vi "生产者消费者.vi"() -> ()   [LabVIEW 2013] (continued)
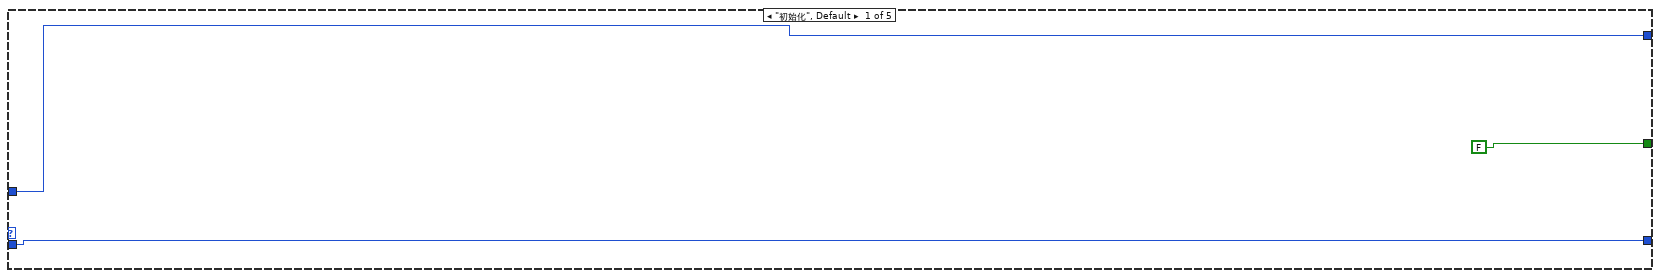
[diagram p2: hidden frame]
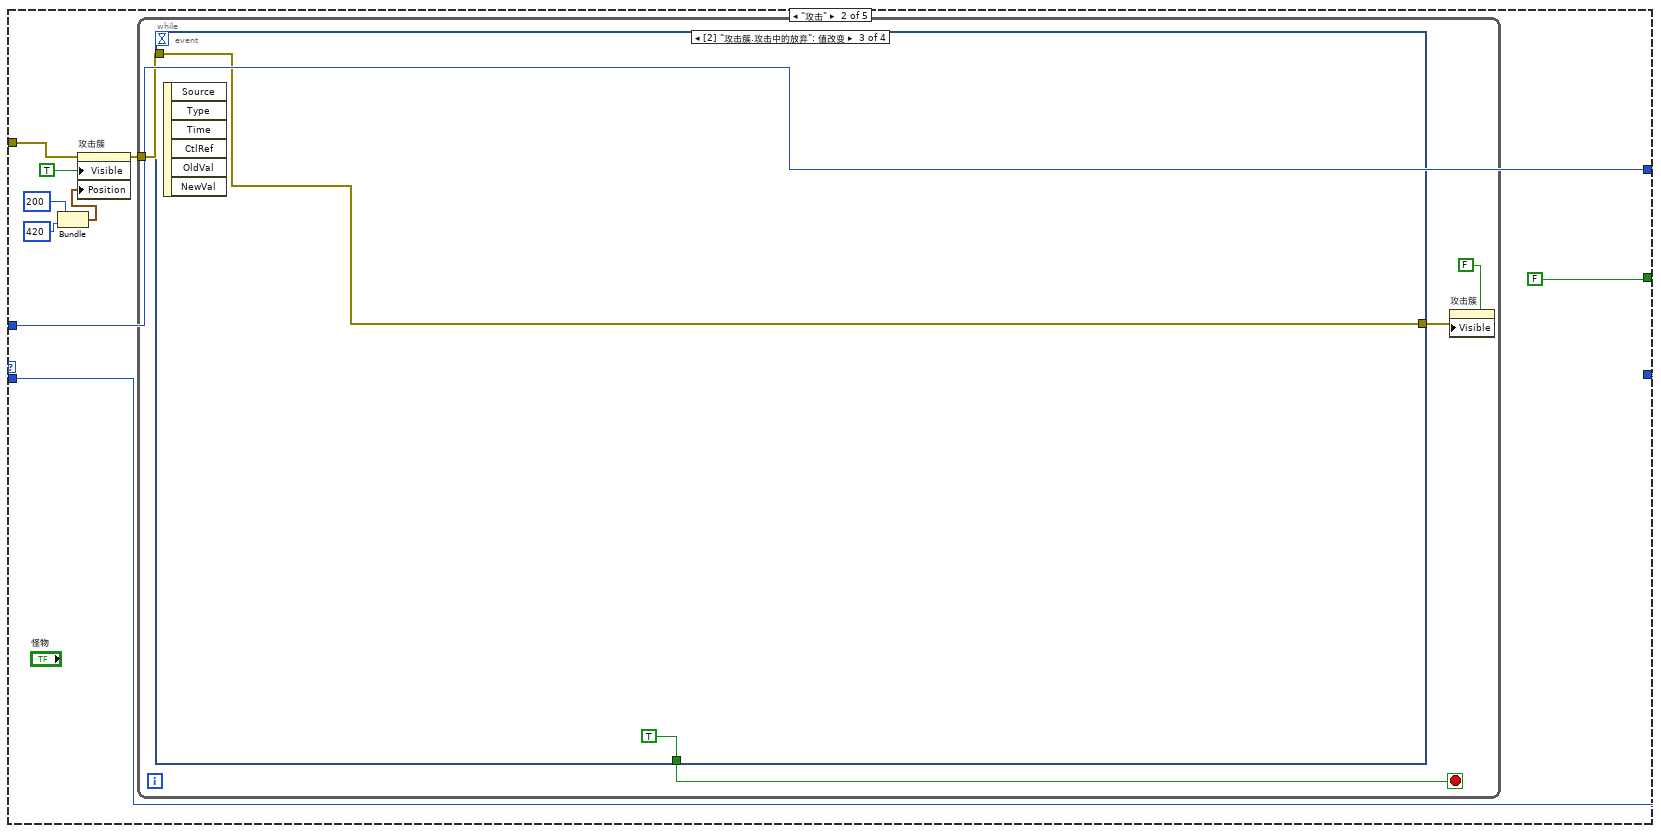
[diagram p3: hidden frame]
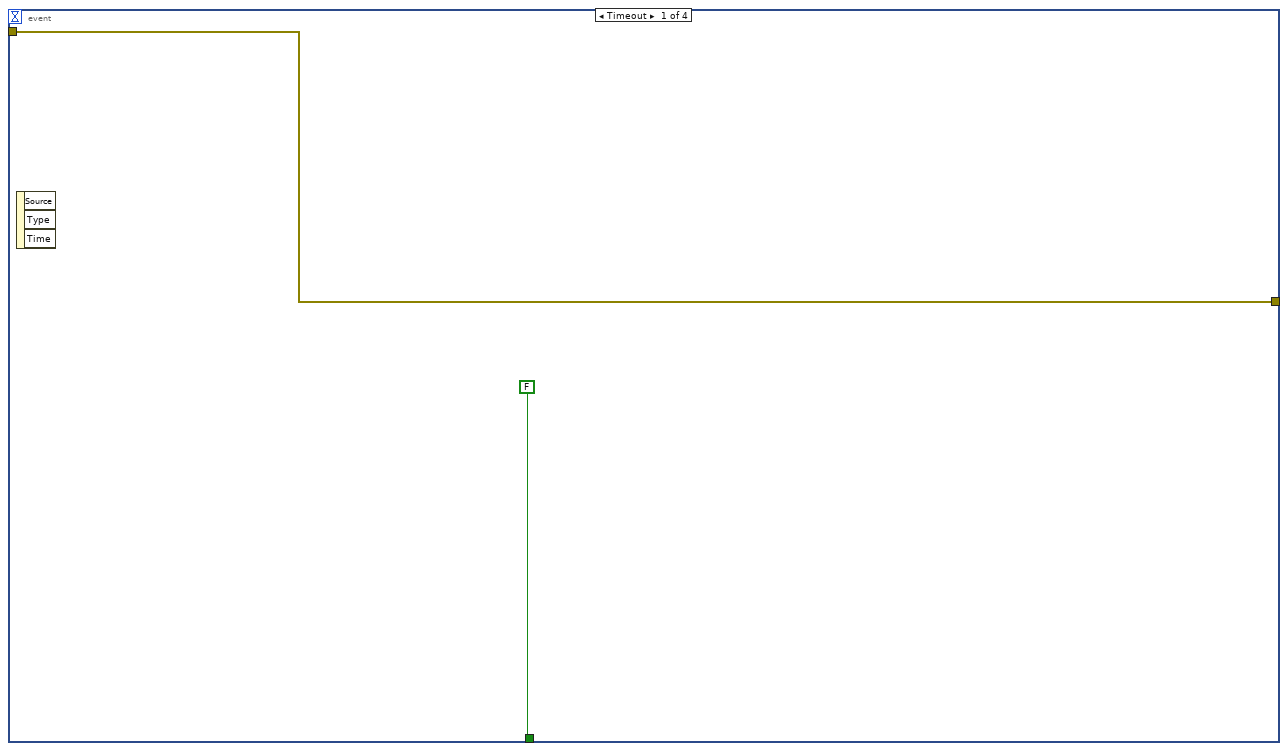
[diagram p4: hidden frame]
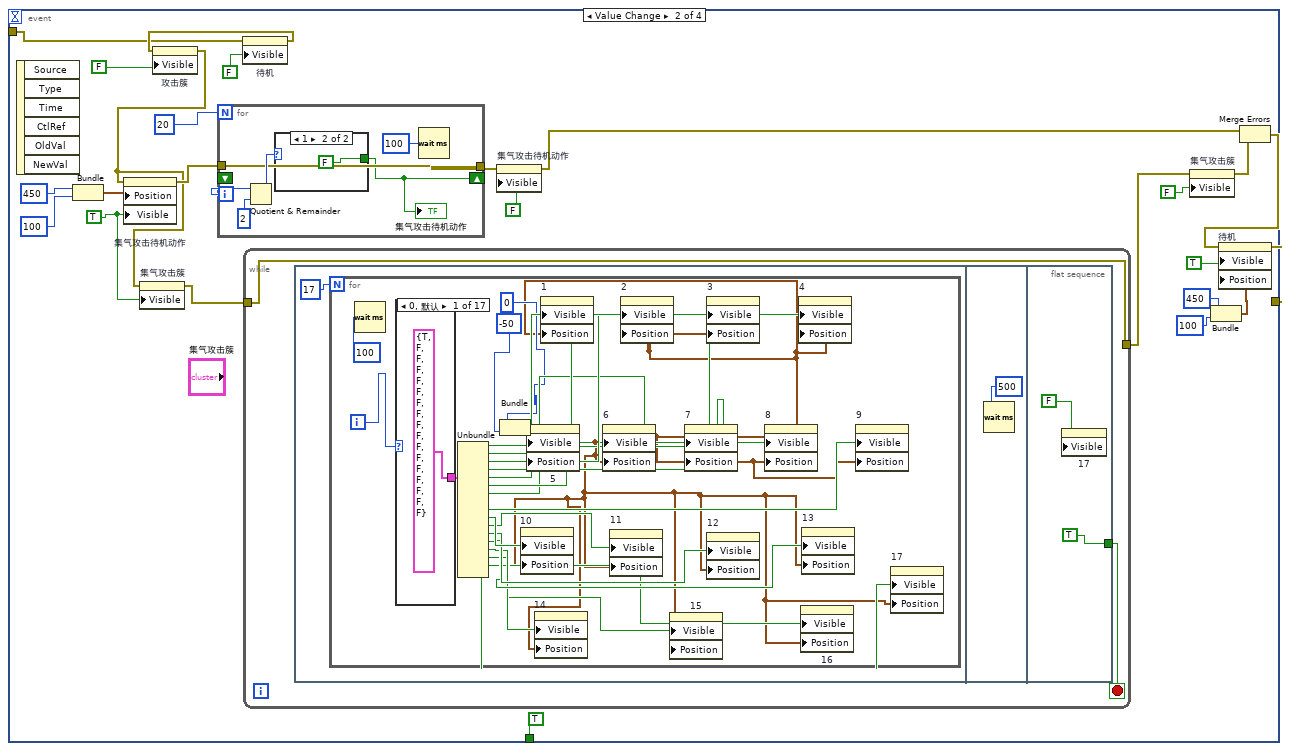
[diagram p5: hidden frame]
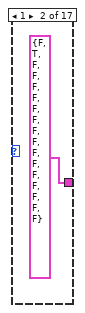
[diagram p6: hidden frame]
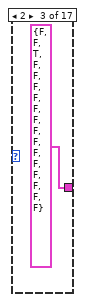
[diagram p7: hidden frame]
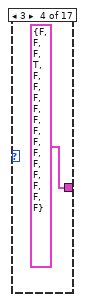
[diagram p8: hidden frame]
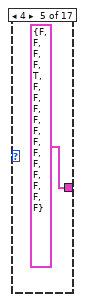
[diagram p9: hidden frame]
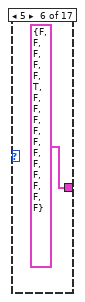
[diagram p10: hidden frame]
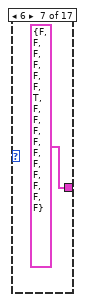
[diagram p11: hidden frame]
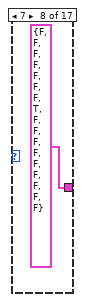
[diagram p12: hidden frame]
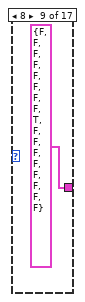
[diagram p13: hidden frame]
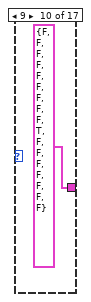
[diagram p14: hidden frame]
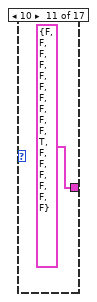
[diagram p15: hidden frame]
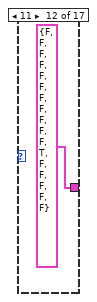
[diagram p16: hidden frame]
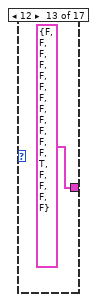
[diagram p17: hidden frame]
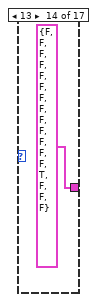
[diagram p18: hidden frame]
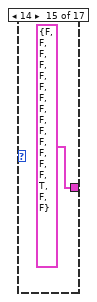
[diagram p19: hidden frame]
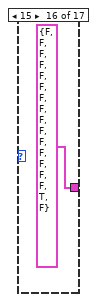
[diagram p20: hidden frame]
                      }
                      frame #2 {
                        n118 = property on="确定按钮" class="Bool"("Visible"=FALSE) -> ()  [unwired: 2 in, 2 out]
                        n119 = property on="15" class="Bool"("Visible"=FALSE) -> ()  [unwired: 2 in, 2 out]
                      }
                    }
                  }
                  n120 = property on="火爪术簇" class="Clust"(error in=w187, "Visible"=FALSE ("可见")) -> ()  [unwired: 1 in, 2 out]
                }
                event "仙术簇.凝冰术": Value Change {
                  n121 = event-data() -> ()  [unwired: 1 in, 6 out]
                  n122 = Bundle(0, 0) -> (w248:cluster{i32, i32})  [unwired: 1 in]
                  n123 = property on="仙术簇" class="Clust"(error in=w251, "Visible"=FALSE) -> (error out=w254:errorcluster)  [unwired: 1 in, 1 out]
                  n124 = property on="待机" class="Bool"(error in=w254, "Visible"=TRUE) -> (error out=w252:errorcluster)  [unwired: 1 in, 1 out]
                  n125 = property on="凝冰术簇" class="Clust"(error in=w252, "Visible"=TRUE, "Position"=w248) -> (error out=w245:errorcluster)  [unwired: 1 in, 1 out]
                  n126 = while {
                    tunnel: w245 -> [w257]
                    tunnel: [w257] -> w244
                    stop <- w258 stop-if-true
                    n127 = flat-sequence {
                      tunnel: [TRUE] -> w258
                      frame #0 {
                        n128 = for {
                          N: 15 -> [_]
                          i -> [w270]
                          n129 = Wait (ms)(milliseconds to wait=100) -> ()  [unwired: 1 out]
                          n130 = case shown="14" w270 {
                            tunnel: [T3 {"4"=TRUE, "5"=FALSE, "6"=FALSE, "7"=FALSE, "8"=FALSE, "1"=FALSE, "2"=FALSE, "3"=FALSE, "9"=FALSE, "10"=FALSE, "11"=FALSE, "12"=FALSE, "13"=FALSE, "14"=FALSE, "15"=FALSE, "确定按钮"=FALSE} ("簇") T3 {"4"=FALSE, "5"=TRUE, "6"=FALSE, "7"=FALSE, "8"=FALSE, "1"=FALSE, "2"=FALSE, "3"=FALSE, "9"=FALSE, "10"=FALSE, "11"=FALSE, "12"=FALSE, "13"=FALSE, "14"=FALSE, "15"=FALSE, "确定按钮"=FALSE} ("簇") T3 {"4"=FALSE, "5"=FALSE, "6"=TRUE, "7"=FALSE, "8"=FALSE, "1"=FALSE, "2"=FALSE, "3"=FALSE, "9"=FALSE, "10"=FALSE, "11"=FALSE, "12"=FALSE, "13"=FALSE, "14"=FALSE, "15"=FALSE, "确定按钮"=FALSE} ("簇") T3 {"4"=FALSE, "5"=FALSE, "6"=FALSE, "7"=TRUE, "8"=FALSE, "1"=FALSE, "2"=FALSE, "3"=FALSE, "9"=FALSE, "10"=FALSE, "11"=FALSE, "12"=FALSE, "13"=FALSE, "14"=FALSE, "15"=FALSE, "确定按钮"=FALSE} ("簇") T3 {"4"=FALSE, "5"=FALSE, "6"=FALSE, "7"=FALSE, "8"=TRUE, "1"=FALSE, "2"=FALSE, "3"=FALSE, "9"=FALSE, "10"=FALSE, "11"=FALSE, "12"=FALSE, "13"=FALSE, "14"=FALSE, "15"=FALSE, "确定按钮"=FALSE} ("簇") T3 {"4"=FALSE, "5"=FALSE, "6"=FALSE, "7"=FALSE, "8"=FALSE, "1"=TRUE, "2"=FALSE, "3"=FALSE, "9"=FALSE, "10"=FALSE, "11"=FALSE, "12"=FALSE, "13"=FALSE, "14"=FALSE, "15"=FALSE, "确定按钮"=FALSE} ("簇") T3 {"4"=FALSE, "5"=FALSE, "6"=FALSE, "7"=FALSE, "8"=FALSE, "1"=FALSE, "2"=TRUE, "3"=FALSE, "9"=FALSE, "10"=FALSE, "11"=FALSE, "12"=FALSE, "13"=FALSE, "14"=FALSE, "15"=FALSE, "确定按钮"=FALSE} ("簇") T3 {"4"=FALSE, "5"=FALSE, "6"=FALSE, "7"=FALSE, "8"=FALSE, "1"=FALSE, "2"=FALSE, "3"=TRUE, "9"=FALSE, "10"=FALSE, "11"=FALSE, "12"=FALSE, "13"=FALSE, "14"=FALSE, "15"=FALSE, "确定按钮"=FALSE} ("簇") T3 {"4"=FALSE, "5"=FALSE, "6"=FALSE, "7"=FALSE, "8"=FALSE, "1"=FALSE, "2"=FALSE, "3"=FALSE, "9"=TRUE, "10"=FALSE, "11"=FALSE, "12"=FALSE, "13"=FALSE, "14"=FALSE, "15"=FALSE, "确定按钮"=FALSE} ("簇") T3 {"4"=FALSE, "5"=FALSE, "6"=FALSE, "7"=FALSE, "8"=FALSE, "1"=FALSE, "2"=FALSE, "3"=FALSE, "9"=FALSE, "10"=TRUE, "11"=FALSE, "12"=FALSE, "13"=FALSE, "14"=FALSE, "15"=FALSE, "确定按钮"=FALSE} ("簇") T3 {"4"=FALSE, "5"=FALSE, "6"=FALSE, "7"=FALSE, "8"=FALSE, "1"=FALSE, "2"=FALSE, "3"=FALSE, "9"=FALSE, "10"=FALSE, "11"=TRUE, "12"=FALSE, "13"=FALSE, "14"=FALSE, "15"=FALSE, "确定按钮"=FALSE} ("簇") T3 {"4"=FALSE, "5"=FALSE, "6"=FALSE, "7"=FALSE, "8"=FALSE, "1"=FALSE, "2"=FALSE, "3"=FALSE, "9"=FALSE, "10"=FALSE, "11"=FALSE, "12"=TRUE, "13"=FALSE, "14"=FALSE, "15"=FALSE, "确定按钮"=FALSE} ("簇") T3 {"4"=FALSE, "5"=FALSE, "6"=FALSE, "7"=FALSE, "8"=FALSE, "1"=FALSE, "2"=FALSE, "3"=FALSE, "9"=FALSE, "10"=FALSE, "11"=FALSE, "12"=FALSE, "13"=TRUE, "14"=FALSE, "15"=FALSE, "确定按钮"=FALSE} ("簇") T3 {"4"=FALSE, "5"=FALSE, "6"=FALSE, "7"=FALSE, "8"=FALSE, "1"=FALSE, "2"=FALSE, "3"=FALSE, "9"=FALSE, "10"=FALSE, "11"=FALSE, "12"=FALSE, "13"=FALSE, "14"=TRUE, "15"=FALSE, "确定按钮"=FALSE} ("簇") T3 {"4"=FALSE, "5"=FALSE, "6"=FALSE, "7"=FALSE, "8"=FALSE, "1"=FALSE, "2"=FALSE, "3"=FALSE, "9"=FALSE, "10"=FALSE, "11"=FALSE, "12"=FALSE, "13"=FALSE, "14"=FALSE, "15"=TRUE, "确定按钮"=FALSE} ("簇")] -> w269
                            frame 0, Default {
                            }
                            frame 1 {
                            }
                            frame 2 {
                            }
                            frame 3 {
                            }
                            frame 4 {
                            }
                            frame 5 {
                            }
                            frame 6 {
                            }
                            frame 7 {
                            }
                            frame 8 {
                            }
                            frame 9 {
                            }
                            frame 10 {
                            }
                            frame 11 {
                            }
                            frame 12 {
                            }
                            frame 13 {
                            }
                            frame 14 {
                            }
                          }
                          n131 = Unbundle(w269) -> ("4"=w282:bool, "5"=w281:bool, "6"=w280:bool, "7"=w279:bool, "8"=w278:bool, "1"=w277:bool, "2"=w265:bool, "3"=w264:bool, "9"=w274:bool, "10"=w273:bool, "11"=w268:bool, "12"=w272:bool, "13"=w262:bool, "14"=w263:bool, "15"=w260:bool)  [unwired: 1 out]
                          n132 = Bundle(50, 0) -> (w271:cluster{i32, i32})  [unwired: 1 in]
                          n133 = property on="确定按钮 10" class="Bool"("Visible"=w273, "Position"=w271) -> ()  [unwired: 2 in, 2 out]
                          n134 = property on="确定按钮 5" class="Bool"("Visible"=w278, "Position"=w271) -> ()  [unwired: 2 in, 2 out]
                          n135 = property on="确定按钮 14" class="Bool"("Visible"=w263, "Position"=w271) -> ()  [unwired: 2 in, 2 out]
                          n136 = property on="确定按钮1" class="Bool"("Visible"=w282, "Position"=w271) -> ()  [unwired: 2 in, 2 out]
                          n137 = property on="确定按钮 6" class="Bool"("Visible"=w277, "Position"=w271) -> ()  [unwired: 2 in, 2 out]
                          n138 = property on="确定按钮 11" class="Bool"("Visible"=w268, "Position"=w271) -> ()  [unwired: 2 in, 2 out]
                          n139 = property on="确定按钮 2" class="Bool"("Visible"=w281, "Position"=w271) -> ()  [unwired: 2 in, 2 out]
                          n140 = property on="确定按钮 15" class="Bool"("Visible"=w260, "Position"=w271) -> ()  [unwired: 2 in, 2 out]
                          n141 = property on="确定按钮 7" class="Bool"("Visible"=w265, "Position"=w271) -> ()  [unwired: 2 in, 2 out]
                          n142 = property on="确定按钮 3" class="Bool"("Visible"=w280, "Position"=w271) -> ()  [unwired: 2 in, 2 out]
                          n143 = property on="确定按钮 12" class="Bool"("Visible"=w272, "Position"=w271) -> ()  [unwired: 2 in, 2 out]
                          n144 = property on="确定按钮 8" class="Bool"("Visible"=w264, "Position"=w271) -> ()  [unwired: 2 in, 2 out]
                          n145 = Bundle(100, 50) -> (w261:cluster{i32, i32})  [unwired: 1 in]
                          n146 = property on="确定按钮 4" class="Bool"("Visible"=w279, "Position"=w271) -> ()  [unwired: 2 in, 2 out]
                          n147 = property on="确定按钮 13" class="Bool"("Visible"=w262, "Position"=w271) -> ()  [unwired: 2 in, 2 out]
                          n148 = property class="Bool"("Visible"=w260, "Position"=w261) -> ()  [unwired: 2 in, 2 out]
                          n149 = property on="确定按钮 9" class="Bool"("Visible"=w274, "Position"=w271) -> ()  [unwired: 2 in, 2 out]
                        }
                      }
                      frame #1 {
                        n150 = Wait (ms)(milliseconds to wait=500) -> ()  [unwired: 1 out]
                      }
                      frame #2 {
                        n151 = property on="确定按钮 15" class="Bool"("Visible"=FALSE) -> ()  [unwired: 2 in, 2 out]
                        n152 = property class="Bool"("Visible"=FALSE) -> ()  [unwired: 2 in, 2 out]
                      }
                    }
                  }
                  n153 = property on="凝冰术簇" class="Clust"(error in=w244, "Visible"=FALSE ("可见")) -> ()  [unwired: 1 in, 2 out]
                }
                event "仙术簇.疾风术": Value Change {
                  n154 = event-data() -> ()  [unwired: 1 in, 6 out]
                  n155 = Bundle(0, 0) -> (w307:cluster{i32, i32})  [unwired: 1 in]
                  n156 = property on="仙术簇" class="Clust"(error in=w310, "Visible"=FALSE) -> (error out=w313:errorcluster)  [unwired: 1 in, 1 out]
                  n157 = property on="待机" class="Bool"(error in=w313, "Visible"=TRUE) -> (error out=w311:errorcluster)  [unwired: 1 in, 1 out]
                  n158 = property on="疾风术簇" class="Clust"(error in=w311, "Visible"=TRUE, "Position"=w307) -> (error out=w304:errorcluster)  [unwired: 1 in, 1 out]
                  n159 = while {
                    tunnel: w304 -> [w316]
                    tunnel: [w316] -> w303
                    stop <- w317 stop-if-true
                    n160 = flat-sequence {
                      tunnel: [TRUE] -> w317
                      frame #0 {
                        n161 = for {
                          N: 14 -> [_]
                          i -> [w330]
                          n162 = Wait (ms)(milliseconds to wait=100) -> ()  [unwired: 1 out]
                          n163 = case shown="13" w330 {
                            tunnel: [T3 {"4"=TRUE, "5"=FALSE, "6"=FALSE, "7"=FALSE, "8"=FALSE, "1"=FALSE, "2"=FALSE, "3"=FALSE, "9"=FALSE, "10"=FALSE, "11"=FALSE, "12"=FALSE, "13"=FALSE, "14"=FALSE, "15"=FALSE, "确定按钮"=FALSE} ("簇") T3 {"4"=FALSE, "5"=TRUE, "6"=FALSE, "7"=FALSE, "8"=FALSE, "1"=FALSE, "2"=FALSE, "3"=FALSE, "9"=FALSE, "10"=FALSE, "11"=FALSE, "12"=FALSE, "13"=FALSE, "14"=FALSE, "15"=FALSE, "确定按钮"=FALSE} ("簇") T3 {"4"=FALSE, "5"=FALSE, "6"=TRUE, "7"=FALSE, "8"=FALSE, "1"=FALSE, "2"=FALSE, "3"=FALSE, "9"=FALSE, "10"=FALSE, "11"=FALSE, "12"=FALSE, "13"=FALSE, "14"=FALSE, "15"=FALSE, "确定按钮"=FALSE} ("簇") T3 {"4"=FALSE, "5"=FALSE, "6"=FALSE, "7"=TRUE, "8"=FALSE, "1"=FALSE, "2"=FALSE, "3"=FALSE, "9"=FALSE, "10"=FALSE, "11"=FALSE, "12"=FALSE, "13"=FALSE, "14"=FALSE, "15"=FALSE, "确定按钮"=FALSE} ("簇") T3 {"4"=FALSE, "5"=FALSE, "6"=FALSE, "7"=FALSE, "8"=TRUE, "1"=FALSE, "2"=FALSE, "3"=FALSE, "9"=FALSE, "10"=FALSE, "11"=FALSE, "12"=FALSE, "13"=FALSE, "14"=FALSE, "15"=FALSE, "确定按钮"=FALSE} ("簇") T3 {"4"=FALSE, "5"=FALSE, "6"=FALSE, "7"=FALSE, "8"=FALSE, "1"=TRUE, "2"=FALSE, "3"=FALSE, "9"=FALSE, "10"=FALSE, "11"=FALSE, "12"=FALSE, "13"=FALSE, "14"=FALSE, "15"=FALSE, "确定按钮"=FALSE} ("簇") T3 {"4"=FALSE, "5"=FALSE, "6"=FALSE, "7"=FALSE, "8"=FALSE, "1"=FALSE, "2"=TRUE, "3"=FALSE, "9"=FALSE, "10"=FALSE, "11"=FALSE, "12"=FALSE, "13"=FALSE, "14"=FALSE, "15"=FALSE, "确定按钮"=FALSE} ("簇") T3 {"4"=FALSE, "5"=FALSE, "6"=FALSE, "7"=FALSE, "8"=FALSE, "1"=FALSE, "2"=FALSE, "3"=TRUE, "9"=FALSE, "10"=FALSE, "11"=FALSE, "12"=FALSE, "13"=FALSE, "14"=FALSE, "15"=FALSE, "确定按钮"=FALSE} ("簇") T3 {"4"=FALSE, "5"=FALSE, "6"=FALSE, "7"=FALSE, "8"=FALSE, "1"=FALSE, "2"=FALSE, "3"=FALSE, "9"=TRUE, "10"=FALSE, "11"=FALSE, "12"=FALSE, "13"=FALSE, "14"=FALSE, "15"=FALSE, "确定按钮"=FALSE} ("簇") T3 {"4"=FALSE, "5"=FALSE, "6"=FALSE, "7"=FALSE, "8"=FALSE, "1"=FALSE, "2"=FALSE, "3"=FALSE, "9"=FALSE, "10"=TRUE, "11"=FALSE, "12"=FALSE, "13"=FALSE, "14"=FALSE, "15"=FALSE, "确定按钮"=FALSE} ("簇") T3 {"4"=FALSE, "5"=FALSE, "6"=FALSE, "7"=FALSE, "8"=FALSE, "1"=FALSE, "2"=FALSE, "3"=FALSE, "9"=FALSE, "10"=FALSE, "11"=TRUE, "12"=FALSE, "13"=FALSE, "14"=FALSE, "15"=FALSE, "确定按钮"=FALSE} ("簇") T3 {"4"=FALSE, "5"=FALSE, "6"=FALSE, "7"=FALSE, "8"=FALSE, "1"=FALSE, "2"=FALSE, "3"=FALSE, "9"=FALSE, "10"=FALSE, "11"=FALSE, "12"=TRUE, "13"=FALSE, "14"=FALSE, "15"=FALSE, "确定按钮"=FALSE} ("簇") T3 {"4"=FALSE, "5"=FALSE, "6"=FALSE, "7"=FALSE, "8"=FALSE, "1"=FALSE, "2"=FALSE, "3"=FALSE, "9"=FALSE, "10"=FALSE, "11"=FALSE, "12"=FALSE, "13"=TRUE, "14"=FALSE, "15"=FALSE, "确定按钮"=FALSE} ("簇") T3 {"4"=FALSE, "5"=FALSE, "6"=FALSE, "7"=FALSE, "8"=FALSE, "1"=FALSE, "2"=FALSE, "3"=FALSE, "9"=FALSE, "10"=FALSE, "11"=FALSE, "12"=FALSE, "13"=FALSE, "14"=TRUE, "15"=FALSE, "确定按钮"=FALSE} ("簇")] -> w329
                            frame 0, Default {
                            }
                            frame 1 {
                            }
                            frame 2 {
                            }
                            frame 3 {
                            }
                            frame 4 {
                            }
                            frame 5 {
                            }
                            frame 6 {
                            }
                            frame 7 {
                            }
                            frame 8 {
                            }
                            frame 9 {
                            }
                            frame 10 {
                            }
                            frame 11 {
                            }
                            frame 12 {
                            }
                            frame 13 {
                            }
                          }
                          n164 = Unbundle(w329) -> ("4"=w341:bool, "5"=w340:bool, "6"=w339:bool, "7"=w338:bool, "8"=w337:bool, "1"=w336:bool, "2"=w326:bool, "3"=w325:bool, "9"=w333:bool, "10"=w332:bool, "11"=w323:bool, "12"=w322:bool, "13"=w321:bool, "14"=w320:bool)  [unwired: 2 out]
                          n165 = Bundle(50, 0) -> (w331:cluster{i32, i32})  [unwired: 1 in]
                          n166 = property on="确定按钮 10" class="Bool"("Visible"=w332, "Position"=w331) -> ()  [unwired: 2 in, 2 out]
                          n167 = property on="确定按钮 5" class="Bool"("Visible"=w337, "Position"=w331) -> ()  [unwired: 2 in, 2 out]
                          n168 = property on="确定按钮 14" class="Bool"("Visible"=w320, "Position"=w331) -> ()  [unwired: 2 in, 2 out]
                          n169 = property on="确定按钮" class="Bool"("Visible"=w341, "Position"=w331) -> ()  [unwired: 2 in, 2 out]
                          n170 = property on="确定按钮 6" class="Bool"("Visible"=w336, "Position"=w331) -> ()  [unwired: 2 in, 2 out]
                          n171 = property on="确定按钮 11" class="Bool"("Visible"=w323, "Position"=w331) -> ()  [unwired: 2 in, 2 out]
                          n172 = property on="确定按钮 2" class="Bool"("Visible"=w340, "Position"=w331) -> ()  [unwired: 2 in, 2 out]
                          n173 = Compound Arithmetic op=OR(w323, w322, w321, w320) -> (w319:bool)
                          n174 = property on="确定按钮 7" class="Bool"("Visible"=w326, "Position"=w331) -> ()  [unwired: 2 in, 2 out]
                          n175 = property on="确定按钮 3" class="Bool"("Visible"=w339, "Position"=w331) -> ()  [unwired: 2 in, 2 out]
                          n176 = property on="确定按钮 12" class="Bool"("Visible"=w322, "Position"=w331) -> ()  [unwired: 2 in, 2 out]
                          n177 = property on="确定按钮 8" class="Bool"("Visible"=w325, "Position"=w331) -> ()  [unwired: 2 in, 2 out]
                          n178 = Bundle(50, 50) -> (w324:cluster{i32, i32})  [unwired: 1 in]
                          n179 = property on="确定按钮 4" class="Bool"("Visible"=w338, "Position"=w331) -> ()  [unwired: 2 in, 2 out]
                          n180 = property on="确定按钮 13" class="Bool"("Visible"=w321, "Position"=w331) -> ()  [unwired: 2 in, 2 out]
                          n181 = property on="确定按钮 15" class="Bool"("Visible"=w319, "Position"=w324) -> ()  [unwired: 2 in, 2 out]
                          n182 = property on="确定按钮 9" class="Bool"("Visible"=w333, "Position"=w331) -> ()  [unwired: 2 in, 2 out]
                        }
                      }
                      frame #1 {
                        n183 = Wait (ms)(milliseconds to wait=500) -> ()  [unwired: 1 out]
                      }
                      frame #2 {
                        n184 = property on="确定按钮 14" class="Bool"("Visible"=FALSE) -> ()  [unwired: 2 in, 2 out]
                        n185 = property on="确定按钮 15" class="Bool"("Visible"=FALSE) -> ()  [unwired: 2 in, 2 out]
                      }
                    }
                  }
                  n186 = property on="疾风术簇" class="Clust"(error in=w303, "Visible"=FALSE ("可见")) -> ()  [unwired: 1 in, 2 out]
                }
                event "仙术簇.仙术中的放弃": Value Change {
                  n187 = event-data() -> ()  [unwired: 1 in, 6 out]
                  n188 = property on="仙术簇" class="Clust"(error in=w361, "Visible"=FALSE) -> ()  [unwired: 1 in, 2 out]
                }
              }
            }
          }
          frame "物品" {
            w366 = FALSE
            n189 = Bundle(200, 420) -> (w375:cluster{i32, i32})  [unwired: 1 in]
            n190 = property on="物品簇" class="Clust"(error in=w379, "Visible"=TRUE, "Position"=w375) -> (error out=w378:errorcluster)  [unwired: 1 in, 1 out]
            n191 = while {
              tunnel: w378 -> [w386]
              tunnel: w374 -> [w385]
              tunnel: [w382] -> w373
              tunnel: [w384] -> w369
              tunnel: w368 -> [w383]
              tunnel: [w381] -> w367
              stop <- w387 stop-if-true
              n192 = event shown="[1] \"物品簇.止血草\": 鼠标进入" {
                selector: _ -> [_ _ _ _ _ _ _]
                dyn-events: _ -> [_ _ _ _ _ _ _]
                timeout: _ -> [_ _ _ _ _ _ _]
                tunnel: [w390 w392 w407 w416 w429 w440 w444] -> w384
                tunnel: [FALSE FALSE FALSE TRUE TRUE TRUE FALSE] -> w387
                tunnel: w386 -> [w390 w402 w413 w416 w429 w440 w442]
                tunnel: w385 -> [w389 w397 w408 w417 w427 w439 w443]
                tunnel: [w389 w397 w408 w418 w427 w439 w443] -> w382
                tunnel: w383 -> [w388 w396 w406 w415 w428 w437 w441]
                tunnel: [w388 w396 w406 w415 w426 w437 w441] -> w381
                event Timeout {
                  n193 = event-data() -> ()  [unwired: 1 in, 3 out]
                }
                event "物品簇.止血草": Mouse Enter {
                  (unwired) 10
                  n194 = event-data() -> ()  [unwired: 1 in, 4 out]
                  n195 = Bundle(400, 200) -> (w398:cluster{i32, i32})  [unwired: 1 in]
                  n196 = property on="琉璃法珠簇" class="Clust"(error in=w402, "Visible"=TRUE, "Position"=w398) -> (error out=w395:errorcluster)  [unwired: 1 in, 1 out]
                  n197 = flat-sequence {
                    tunnel: w395 -> [w404]
                    tunnel: [w404] -> w393
                    frame #0 {
                      n198 = Wait (ms)(milliseconds to wait=1000) -> ()  [unwired: 1 out]
                    }
                  }
                  n199 = property on="琉璃法珠簇" class="Clust"(error in=w393, "Visible"=FALSE) -> (error out=w392:errorcluster)  [unwired: 1 in, 1 out]
                }
                event "物品簇.鼠儿果": Mouse Enter {
                  (unwired) 10
                  n200 = event-data() -> ()  [unwired: 1 in, 4 out]
                  n201 = Bundle(400, 200) -> (w409:cluster{i32, i32})  [unwired: 1 in]
                  n202 = property on="龙蟠雕玉" class="Clust"(error in=w413, "Visible"=TRUE, "Position"=w409) -> (error out=w407:errorcluster)  [unwired: 1 in, 1 out]
                }
                event "物品簇.止血草": Value Change {
                  n203 = event-data() -> ()  [unwired: 1 in, 6 out]
                  n204 = Greater?(x=w417, y=100) -> (0:w419:bool)
                  n205 = case shown="真" w419 {
                    tunnel: [w422 200] -> w418
                    tunnel: w417 -> [w424 _]
                    frame False {
                      n206 = Add(x=w424, y=100) -> (x+y=w422:i32)
                    }
                    frame True {
                    }
                  }
                }
                event "物品簇.鼠儿果": Value Change {
                  n207 = event-data() -> ()  [unwired: 1 in, 6 out]
                  n208 = Greater?(x=w428, y=100) -> (0:w430:bool)
                  n209 = case shown="真" w430 {
                    tunnel: [w434 200] -> w426
                    tunnel: w428 -> [w433 _]
                    frame False {
                      n210 = Add(x=w433, y=100) -> (x+y=w434:i32)
                    }
                    frame True {
                    }
                  }
                }
                event "物品簇.物品中的放弃": Value Change {
                  n211 = event-data() -> ()  [unwired: 1 in, 6 out]
                }
                event "物品簇.鼠儿果": Mouse Leave {
                  n212 = event-data() -> ()  [unwired: 1 in, 4 out]
                  n213 = property on="龙蟠雕玉" class="Clust"(error in=w442, "Visible"=FALSE) -> (error out=w444:errorcluster)  [unwired: 1 in, 1 out]
                }
              }
            }
            n214 = Bundle(200, 420) -> (w370:cluster{i32, i32})  [unwired: 1 in]
            n215 = property on="物品簇" class="Clust"(error in=w369, "Visible"=w366, "Position"=w370) -> (error out=w365:errorcluster)  [unwired: 1 in, 1 out]
            n216 = property on="龙蟠雕玉" class="Clust"(error in=w365, "Visible"=w366) -> ()  [unwired: 1 in, 2 out]
            n217 = property on="琉璃法珠簇" class="Clust"(error in=w365, "Visible"=w366) -> ()  [unwired: 1 in, 2 out]
          }
          frame "逃跑" {
            n218 = Bundle(200, 140) -> (w449:cluster{i32, i32})  [unwired: 1 in]
            n219 = property on="逃跑成功" class="Bool"(error in=w454, "Visible"=TRUE, "Position"=w449) -> (error out=w448:errorcluster)  [unwired: 1 in, 1 out]
            n220 = flat-sequence {
              tunnel: w448 -> [w456]
              tunnel: [TRUE] -> w447
              tunnel: [w456] -> _
              frame #0 {
                n221 = Wait (ms)(milliseconds to wait=500) -> ()  [unwired: 1 out]
              }
            }
          }
        }
        n222 = Or(x=w18, y=FALSE) -> (x .or. y?=w16:bool)
      }
      frame Error {
      }
    }
  }
  n223 = while {
    shift-right: [w479] -> w6
    shift-left: w7 -> [w472]
    tunnel: w5 -> [w482]
    stop <- w480 stop-if-true
    n224 = Bundle(450, 100) -> (w468:cluster{i32, i32})  [unwired: 1 in]
    n225 = property on="待机" class="Bool"(error in=w472, "Visible"=TRUE, "Position"=w468) -> (error out=w467:errorcluster)  [unwired: 1 in, 1 out]
    n226 = property on="逃跑成功" class="Bool"(error in=w467, "Visible"=FALSE ("可见")) -> (error out=w466:errorcluster)  [unwired: 1 in, 1 out]
    n227 = event shown="[2] \"物品\": 值改变" {
      selector: _ -> [_ _ _ _]
      dyn-events: _ -> [_ _ _ _]
      timeout: _ -> [_ _ _ _]
      tunnel: w482 -> [w490 w499 w505 w511]
      tunnel: w466 -> [w489 w498 w504 w510]
      tunnel: [w483 w496 w502 w508] -> w479
      tunnel: [_ TRUE _ _] -> w481
      tunnel: [cluster{bool, bool, bool, bool} {TRUE, FALSE, FALSE, FALSE} cluster{bool, bool, bool, bool} {FALSE, FALSE, FALSE, FALSE} cluster{bool, bool, bool, bool} {FALSE, TRUE, FALSE, FALSE} cluster{bool, bool, bool, bool} {FALSE, FALSE, TRUE, FALSE}] -> w477
      event "攻击": Value Change {
        n228 = event-data() -> ()  [unwired: 1 in, 1 out]
        n229 = Enqueue Element(queue=w490, element=enum16{"逃跑", "初始化", "物品", "仙术", "攻击"}."攻击" ("五个状态"), error in (no error)=w489) -> (error out=w486:errorcluster)  [unwired: 1 in, 2 out]
        n230 = property on="集气攻击待机动作" class="Bool"(error in=w486, "Visible"=FALSE) -> (error out=w484:errorcluster)  [unwired: 1 in, 1 out]
        n231 = invoke on="攻击" class="Bool" method="Reinit To Default"(error in=w484) -> (error out=w483:errorcluster)  [unwired: 2 in, 2 out]
      }
      event "逃跑": Value Change {
        n232 = event-data() -> ()  [unwired: 1 in, 1 out]
        n233 = Enqueue Element(queue=w499, element=enum16{"逃跑", "初始化", "物品", "仙术", "攻击"}."逃跑" ("五个状态"), error in (no error)=w498) -> (error out=w493:errorcluster)  [unwired: 1 in, 2 out]
        n234 = property on="集气攻击待机动作" class="Bool"(error in=w493, "Visible"=FALSE) -> (error out=w495:errorcluster)  [unwired: 1 in, 1 out]
        n235 = invoke on="逃跑" class="Bool" method="Reinit To Default"(error in=w495) -> (error out=w496:errorcluster)  [unwired: 2 in, 2 out]
      }
      event "物品": Value Change {
        n236 = event-data() -> ()  [unwired: 1 in, 1 out]
        n237 = Enqueue Element(queue=w505, element=enum16{"逃跑", "初始化", "物品", "仙术", "攻击"}."物品" ("五个状态"), error in (no error)=w504) -> (error out=w501:errorcluster)  [unwired: 1 in, 2 out]
        n238 = invoke on="物品" class="Bool" method="Reinit To Default"(error in=w501) -> (error out=w502:errorcluster)  [unwired: 2 in, 2 out]
      }
      event "仙术": Value Change {
        n239 = event-data() -> ()  [unwired: 1 in, 1 out]
        n240 = Enqueue Element(queue=w511, element=enum16{"逃跑", "初始化", "物品", "仙术", "攻击"}."仙术" ("五个状态"), error in (no error)=w510) -> (error out=w507:errorcluster)  [unwired: 1 in, 2 out]
        n241 = invoke on="仙术" class="Bool" method="Reinit To Default"(error in=w507) -> (error out=w508:errorcluster)  [unwired: 2 in, 2 out]
      }
    }
    n242 = Unbundle By Name(w479) -> ("status"=w478:bool)
    n243 = Unbundle(w477) -> (w476:bool, w475:bool, w474:bool, w473:bool)
    n244 = property on="集气攻击簇" class="Clust"("Visible"=w473) -> ()  [unwired: 2 in, 2 out]
    n245 = property on="琉璃法珠簇" class="Clust"("Visible"=w473) -> ()  [unwired: 2 in, 2 out]
    n246 = Or(x=w478, y=w481) -> (x .or. y?=w480:bool)
    n247 = Bundle(200, 420) -> (w462:cluster{i32, i32})  [unwired: 1 in]
    n248 = property on="仙术簇" class="Clust"("Visible"=w474, "Position"=w462) -> ()  [unwired: 2 in, 2 out]
    n249 = property on="物品簇" class="Clust"("Visible"=w475, "Position"=w462) -> ()  [unwired: 2 in, 2 out]
    n250 = property on="攻击簇" class="Clust"("Visible"=w476, "Position"=w462) -> ()  [unwired: 2 in, 2 out]
  }
  n251 = Release Queue(queue=w5, error in (no error)=w6) -> ()  [unwired: 1 in, 3 out]
